vi "HFRR ADV v040 new software.vi"() -> ()   [LabVIEW 2025] (continued)
            n2157 = Bundle "Bundle"(w2313, w2312) -> (w2319:cluster{dbl[], dbl[]})  [unwired: 1 in]
            n2158 = Bundle "Bundle"(w2313, w2345) -> (w2456:cluster{dbl[], dbl[]})  [unwired: 1 in]
            n2159 = Bundle "Bundle"(w2313, w2341) -> (w2379:cluster{dbl[], dbl[]})  [unwired: 1 in]
            n2160 = Bundle "Bundle"(w2313, w2395) -> (w2403:cluster{dbl[], dbl[]})  [unwired: 1 in]
            n2161 = Bundle "Bundle"(w2313, w2397) -> (w2465:cluster{dbl[], dbl[]})  [unwired: 1 in]
            n2162 = Bundle "Bundle"(w2313, w2434) -> (w2447:cluster{dbl[], dbl[]})  [unwired: 1 in]
            n2163 = Bundle "Bundle"(w2343, w2339) -> (w2351:cluster{dbl[], dbl[]})  [unwired: 1 in]
            n2164 = Bundle "Bundle"(w2309, w2308) -> (w2317:cluster{dbl[], dbl[]})  [unwired: 1 in]
            n2165 = Bundle "Bundle"(w2309, w2343) -> (w2455:cluster{dbl[], dbl[]})  [unwired: 1 in]
            n2166 = Bundle "Bundle"(w2309, w2339) -> (w2377:cluster{dbl[], dbl[]})  [unwired: 1 in]
            n2167 = Bundle "Bundle"(w2309, w2393) -> (w2401:cluster{dbl[], dbl[]})  [unwired: 1 in]
            n2168 = Bundle "Bundle"(w2309, w2398) -> (w2463:cluster{dbl[], dbl[]})  [unwired: 1 in]
            n2169 = Bundle "Bundle"(w2309, w2416) -> (w2448:cluster{dbl[], dbl[]})  [unwired: 1 in]
            n2170 = call-poly <vilib>:"Mean.vi"("X"=w2396) -> ("mean"=→"CP1":dbl)  [unwired: 1 out]
            n2171 = call-poly <vilib>:"Mean.vi"("X"=w2337) -> ("mean"=→"КОФ2 3":dbl)  [unwired: 1 out]
            n2172 = call-poly <vilib>:"Mean.vi"("X"=w2395) -> ("mean"=→"CP2":dbl)  [unwired: 1 out]
            n2173 = call-poly <vilib>:"Mean.vi"("X"=w2397) -> ("mean"=→"КОФ2":dbl)  [unwired: 1 out]
            n2174 = call-poly <vilib>:"Mean.vi"("X"=w2335) -> ("mean"=→"КОФ2 5":dbl)  [unwired: 1 out]
            n2175 = call-poly <vilib>:"Mean.vi"("X"=w2393) -> ("mean"=→"CP4":dbl)  [unwired: 1 out]
            n2176 = call-poly <vilib>:"Mean.vi"("X"=w2398) -> ("mean"=→"КОФ4":dbl)  [unwired: 1 out]
            n2177 = Bundle "Bundle"(w2315, w2342) -> (w2306:cluster{dbl[], dbl[]})  [unwired: 1 in]
            n2178 = Bundle "Bundle"(w2315, w2396) -> (w2329:cluster{dbl[], dbl[]})  [unwired: 1 in]
            n2179 = Build Array "Build Array"(w2306, w2329) -> (w2332:cluster{dbl[], dbl[]}[])
            "XY Graph 17" <- w2332
            n2180 = Build Array "Build Array"(w2320, w2319, w2318, w2317) -> (→"Frequency ( Hz )":cluster{dbl[], dbl[]}[])
            n2181 = Build Array "Build Array"(w2348, w2349, w2350, w2351) -> (→"Air Temp ( °C ) vs Humidity ( % RH )":cluster{dbl[], dbl[]}[])
            n2182 = Build Array "Build Array"(w2333, w2456, w2454, w2455) -> (→"Air Temperature  ( °C )":cluster{dbl[], dbl[]}[])
            n2183 = Build Array "Build Array"(w2306, w2379, w2378, w2377) -> (→"Humidity ( %RH )":cluster{dbl[], dbl[]}[])
            n2184 = Build Array "Build Array"(w2334, w2465, w2464, w2463) -> (→"Coefficient Of Friction":cluster{dbl[], dbl[]}[])
            n2185 = Build Array "Build Array"(w2329, w2403, w2402, w2401) -> (→"Sample Temperature ( °C )":cluster{dbl[], dbl[]}[])
            n2186 = Build Array "Build Array"(w2307, w2447, w2449, w2448) -> (→"XY Graph 13":cluster{dbl[], dbl[]}[])
            n2187 = Bundle "Bundle"(w2315, w2338) -> (w2360:cluster{dbl[], dbl[]})  [unwired: 1 in]
            n2188 = Bundle "Bundle"(w2311, w2336) -> (w2358:cluster{dbl[], dbl[]})  [unwired: 1 in]
            n2189 = Bundle "Bundle"(w2313, w2337) -> (w2359:cluster{dbl[], dbl[]})  [unwired: 1 in]
            n2190 = Bundle "Bundle"(w2309, w2335) -> (w2357:cluster{dbl[], dbl[]})  [unwired: 1 in]
            n2191 = Build Array "Build Array"(w2360, w2359, w2358, w2357) -> (→"Stroke ( mm )":cluster{dbl[], dbl[]}[])
            n2192 = local write "XY Graph 16"(w2332) -> ()
          }
          frame #2 {
          }
          frame #3 {
            n2193 = local write "Numeric 8"(0 ("Numeric 8")) -> ()
            n2194 = local write "Numeric 11"(0 ("Numeric 11")) -> ()
            n2195 = local write "Numeric 12"(0 ("Numeric 12")) -> ()
            n2196 = local write "Numeric 13"(0 ("Numeric 13")) -> ()
            n2197 = property on="OPEN" class="Bool (strict)"("Visible"=TRUE) -> ()  [unwired: 2 in, 2 out]
            n2198 = local read "String Control 2"() -> (w2632:string)
            n2199 = local read "String Control 4"() -> (w2631:string)
            n2200 = local read "String Control 6"() -> (w2630:string)
            n2201 = local read "String Control 8"() -> (w2629:string)
            n2202 = Match Pattern(string=w2632, regular expression="Samples / cycle :- ") -> (after substring=w2646:string)  [unwired: 1 in, 3 out]
            n2203 = Match Pattern(string=w2632, regular expression="Frequency :- ") -> (after substring=w2665:string)  [unwired: 1 in, 3 out]
            n2204 = Match Pattern(string=w2631, regular expression="Samples / cycle :- ") -> (after substring=w2642:string)  [unwired: 1 in, 3 out]
            n2205 = Match Pattern(string=w2631, regular expression="Frequency :- ") -> (after substring=w2660:string)  [unwired: 1 in, 3 out]
            n2206 = Match Pattern(string=w2630, regular expression="Samples / cycle :- ") -> (after substring=w2638:string)  [unwired: 1 in, 3 out]
            n2207 = Match Pattern(string=w2630, regular expression="Frequency :- ") -> (after substring=w2655:string)  [unwired: 1 in, 3 out]
            n2208 = Match Pattern(string=w2629, regular expression="Samples / cycle :- ") -> (after substring=w2634:string)  [unwired: 1 in, 3 out]
            n2209 = Match Pattern(string=w2629, regular expression="Frequency :- ") -> (after substring=w2650:string)  [unwired: 1 in, 3 out]
            n2210 = String Subset(string=w2646, length (rest)=6 ("length (rest)")) -> (substring=w2648:string)  [unwired: 1 in]
            n2211 = String Subset(string=w2665, length (rest)=9 ("length (rest)")) -> (substring=w2667:string)  [unwired: 1 in]
            n2212 = String Subset(string=w2642, length (rest)=6 ("length (rest)")) -> (substring=w2644:string)  [unwired: 1 in]
            n2213 = String Subset(string=w2660, length (rest)=9 ("length (rest)")) -> (substring=w2662:string)  [unwired: 1 in]
            n2214 = String Subset(string=w2638, length (rest)=6 ("length (rest)")) -> (substring=w2640:string)  [unwired: 1 in]
            n2215 = String Subset(string=w2655, length (rest)=9 ("length (rest)")) -> (substring=w2657:string)  [unwired: 1 in]
            n2216 = String Subset(string=w2634, length (rest)=6 ("length (rest)")) -> (substring=w2636:string)  [unwired: 1 in]
            n2217 = String Subset(string=w2650, length (rest)=9 ("length (rest)")) -> (substring=w2652:string)  [unwired: 1 in]
            n2218 = Fract/Exp String To Number(string=w2648) -> (number=w2628:dbl)  [unwired: 3 in, 1 out]
            n2219 = Fract/Exp String To Number(string=w2667) -> (number=w2668:dbl)  [unwired: 3 in, 1 out]
            n2220 = Fract/Exp String To Number(string=w2644) -> (number=w2627:dbl)  [unwired: 3 in, 1 out]
            n2221 = Fract/Exp String To Number(string=w2662) -> (number=w2663:dbl)  [unwired: 3 in, 1 out]
            n2222 = Fract/Exp String To Number(string=w2640) -> (number=w2626:dbl)  [unwired: 3 in, 1 out]
            n2223 = Fract/Exp String To Number(string=w2657) -> (number=w2658:dbl)  [unwired: 3 in, 1 out]
            n2224 = Fract/Exp String To Number(string=w2636) -> (number=w2625:dbl)  [unwired: 3 in, 1 out]
            n2225 = Fract/Exp String To Number(string=w2652) -> (number=w2653:dbl)  [unwired: 3 in, 1 out]
            n2226 = local write "sample1"(w2628) -> ()
            n2227 = local write "freq1"(w2668) -> ()
            n2228 = local write "sample2"(w2627) -> ()
            n2229 = local write "freq2"(w2663) -> ()
            n2230 = local write "sample3"(w2626) -> ()
            n2231 = local write "freq3"(w2658) -> ()
            n2232 = local write "sample4"(w2625) -> ()
            n2233 = local write "freq 4"(w2653) -> ()
          }
        }
      }
    }
    n2234 = case shown="True" w2226 {
      selector: w2226 -> [_ w2245]
      frame False {
      }
      frame True {
        n2235 = Not(x=w2245) -> (.not. x?=w2241:bool)
        n2236 = local write "service 3"(w2241) -> ()
        n2237 = local write "OPEN 6"(w2241) -> ()
        n2238 = call <vilib>:"System Exec.vi"("wait until completion? (T)"=TRUE, "command line"="C:\\LAB-IQ\\Scar View.exe") -> ("error out"=→"error out 5":errorcluster)  [unwired: 6 in, 3 out]
      }
    }
    n2239 = case shown="\"Acquire\", Default" w2235 {
      frame "Acquire", Default {
        # "Elapsed time\ncof\nstroke\nAir temp\nTemp\nHumidity"
        n2240 = disable-structure shown="Disabled" {
          frame Disabled {
            n2241 = local read "Flag"() -> (w2944:dbl)
            n2242 = local read "RUN"() -> (w2941:bool)
            n2243 = Not(x=w2941) -> (.not. x?=w2940:bool)
            n2244 = Equal?(x=w2944, y=10.0) -> (x = y?=w2942:bool)
            n2245 = And(x=w2942, y=w2940) -> (x .and. y?=w2939:bool)
            n2246 = case shown="True" w2939 {
              frame False {
              }
              frame True {
                w2945 = FALSE ("Heater Button")
                n2247 = local write "Humidity"(w2945) -> ()
                n2248 = local write "Heater Button"(w2945) -> ()
              }
            }
          }
          frame Enabled {
          }
        }
        n2249 = disable-structure shown="Disabled" {
          frame Disabled {
            n2250 = case shown="True" {
              selector: _ -> [_ _]
              frame False {
              }
              frame True {
                w2994 = TRUE ("Heater")
                n2251 = local write "Humidity"(w2994) -> ()
                n2252 = local write "Heater Button"(w2994) -> ()
                n2253 = local read "TEST STANDARD"() -> (w2997:T3)
                n2254 = local read "TEST STANDARD"() -> (w2992:T3)
                n2255 = Equal?(x=w2997, y=enum16{"ASTM D6079", "ISO 12156", "Custom"}."ISO 12156" ("Test Standard")) -> (x = y?=w2995:bool)
                n2256 = Equal?(x=w2992, y=enum16{"ASTM D6079", "ISO 12156", "Custom"}."ASTM D6079" ("Test Standard")) -> (x = y?=w2991:bool)
                n2257 = case shown="True" w2995 {
                  frame False {
                  }
                  frame True {
                    n2258 = local write "airtempflg"(FALSE ("airtempflg")) -> ()
                    n2259 = local write item#-1(TRUE ("Heater")) -> ()
                  }
                }
                n2260 = case shown="True" w2991 {
                  frame False {
                  }
                  frame True {
                    n2261 = local write "airtempflg"(TRUE ("airtempflg")) -> ()
                    n2262 = local write item#-1(FALSE ("Heater")) -> ()
                  }
                }
              }
            }
          }
          frame Enabled {
          }
        }
        n2263 = stacked-sequence {
          frame #0 {
            n2264 = case shown="True" "RST FF" {
              frame False {
              }
              frame True {
                w3011 = 0.0 ("X Scale.Range:Maximum")
                n2265 = property on="Frictional Force ( N )" class="WFChart (strict)"("XScale.Maximum"=600.0 ("X Scale.Range:Maximum"), "XScale.Minimum"=w3011, "YScale.Maximum"=10.0 ("Y Scale.Range:Maximum"), "YScale.Minimum"=w3011) -> ()  [unwired: 2 in, 2 out]
              }
            }
          }
          frame #1 {
            n2266 = case shown="True" "RST TEMP" {
              frame False {
              }
              frame True {
                n2267 = property on="Temperature ( Deg C )" class="WFChart (strict)"("XScale.Minimum"=0.0 ("X Scale.Range:Minimum"), "XScale.Maximum"=600.0 ("X Scale.Range:Maximum"), "YScale.Minimum"=0.0 ("Y Scale.Range:Minimum"), "YScale.Maximum"=100.0 ("Y Scale.Range:Maximum")) -> ()  [unwired: 2 in, 2 out]
              }
            }
          }
          frame #2 {
            n2268 = case shown="True" "RSTCOF" {
              frame False {
              }
              frame True {
                n2269 = property on="Coefficient of Friction" class="WFChart (strict)"("XScale.Minimum"=0.0 ("X Scale.Range:Minimum"), "XScale.Maximum"=600.0 ("X Scale.Range:Maximum"), "YScale.Maximum"=1.0 ("X Scale.Range:Minimum"), "YScale.Minimum"=0.0 ("X Scale.Range:Minimum")) -> ()  [unwired: 2 in, 2 out]
              }
            }
          }
          frame #3 {
            n2270 = case shown="True" "RSTCOF 2" {
              frame False {
              }
              frame True {
                (unwired) 100.0 ("Y Scale.Range:Maximum")
                (unwired) 0.0 ("Y Scale.Range:Minimum")
                (unwired) 600.0 ("X Scale.Range:Maximum")
                (unwired) 0.0 ("X Scale.Range:Minimum")
              }
            }
          }
          frame #4 {
            n2271 = case shown="True" "RSTCOF 3" {
              frame False {
              }
              frame True {
                n2272 = property on="Electrical Contact Resistance ( % )" class="WFChart (strict)"("XScale.Minimum"=0.0 ("X Scale.Range:Minimum"), "XScale.Maximum"=600.0 ("X Scale.Range:Maximum"), "YScale.Minimum"=0.0 ("Y Scale.Range:Minimum"), "YScale.Maximum"=100.0 ("Y Scale.Range:Maximum")) -> ()  [unwired: 2 in, 2 out]
              }
            }
          }
        }
        n2273 = local read "RUN"() -> (w2934:bool)
        n2274 = case shown="False" w2934 {
          frame False {
          }
          frame True {
          }
        }
        n2275 = local read "RUN"() -> (w2938:bool)
        n2276 = case shown="False" w2938 {
          tunnel: [FALSE ("TEST RUNNING") TRUE ("TEST RUNNING")] -> w2937
          frame False {
            w3030 = 0.0 ("Flag")
            n2277 = local write "Elapsed time"(0.0 ("elapsedtime")) -> ()
            n2278 = local write "Time Remaining"(w3030) -> ()
            n2279 = local write "Flag"(w3030) -> ()
            n2280 = local write "Remaining Time"(w3030) -> ()
          }
          frame True {
            n2281 = local write "Flag"(10.0 ("Flag")) -> ()
          }
        }
        n2282 = local read "AIR TEMP"() -> (w2932:dbl)
        n2283 = Greater Or Equal?(x=w2932, y=15.0) -> (x >= y?=w2933:bool)
        "powstat" <- w2933
        n2284 = case shown="True" "Save & Continue" {
          frame False {
          }
          frame True {
            n2285 = local read "USER ID"() -> (w3339:string)
            n2286 = local read "FILE"() -> (w3347:string)
            n2287 = String Length(string=w3347) -> (length=w3345:i32)
            n2288 = String Length(string=w3339) -> (length=w3342:i32)
            n2289 = Greater?(x=w3345, y=0) -> (0:w3344:bool)
            n2290 = Greater?(x=w3342, y=0) -> (0:w3341:bool)
            n2291 = And(x=w3344, y=w3341) -> (x .and. y?=w3340:bool)
            n2292 = case shown="True" w3340 {
              frame False {
                n2293 = stacked-sequence {
                  frame #0 {
                    n2294 = One Button Dialog(message="Please Enter a File Name and Operator ID to save data !", button name ("OK")="Ok") -> ()  [unwired: 1 out]
                  }
                  frame #1 {
                    n2295 = local write "Save & Continue"(FALSE ("OK Button")) -> ()
                  }
                }
                n2296 = local write "Save & Continue"(FALSE ("OK Button")) -> ()
              }
              frame True {
                n2297 = stacked-sequence {
                  frame #0 {
                    n2298 = local read "FILE"() -> (w3353:string)
                    n2299 = call "file check.vi"("file name in"=w3353) -> ("file name out"=w3352:string)  [unwired: 9 in, 1 out]
                    n2300 = call <vilib>:"Application Directory.vi"() -> ("Application Directory"=w3363:path)
                    n2301 = Build Path(base path=w3363, name or relative path="data") -> (appended path=w3362:path)
                    n2302 = call <vilib>:"Trim Whitespace.vi"("string"=w3352) -> ("trimmed string"=w3360:string)  [unwired: 1 in]
                    n2303 = call <vilib>:"Trim Whitespace.vi"("string"=w3352) -> ("trimmed string"=w3361:string)  [unwired: 1 in]
                    n2304 = List Folder(path=w3362) -> (folder names=w3358:string[])  [unwired: 3 in, 3 out]
                    n2305 = Match Pattern(string=w3360, regular expression="_(") -> (before substring=w3357:string)  [unwired: 1 in, 3 out]
                    n2306 = for {
                      tunnel: w3358 -> [w3372] mode=indexing
                      tunnel: w3357 -> [w3370]
                      shift-right: [w3368] -> w3355
                      shift-left: bool[] [] -> [w3369]
                      n2307 = Match Pattern(string=w3372, regular expression="_(") -> (before substring=w3371:string)  [unwired: 1 in, 3 out]
                      n2308 = Equal?(x=w3371, y=w3370) -> (x = y?=w3367:bool)
                      n2309 = case shown="True" w3367 {
                        tunnel: w3367 -> [_ w3375]
                        tunnel: w3369 -> [w3374 w3377]
                        tunnel: [w3374 w3376] -> w3368
                        frame False {
                        }
                        frame True {
                          n2310 = Insert Into Array(array=w3377, new element=w3375) -> (w3376:bool[])  [unwired: 1 in]
                        }
                      }
                    }
                    n2311 = Equal?(x=w3358, y=w3357) -> (x = y?=w3366:bool[])
                    n2312 = Or Array Elements(Boolean array=w3366) -> (logical OR=w3365:bool)
                    n2313 = Array Size(array=w3355) -> (size(s)=w3354:i32)
                    n2314 = case shown="True" w3365 {
                      tunnel: w3361 -> [_ w3385]
                      tunnel: w3354 -> [_ w3378]
                      frame False {
                      }
                      frame True {
                        n2315 = Number To Decimal String(number=w3378) -> (decimal integer string=w3381:string)  [unwired: 1 in]
                        n2316 = Search/Split String(string=w3385, search string/char (-)="_(" ("regular expression")) -> (substring before match=w3383:string)  [unwired: 1 in, 2 out]
                        n2317 = Concatenate Strings(w3383, "_(" ("regular expression"), w3381, ")" ("regular expression")) -> (w3379:string)
                        n2318 = local write "FILE"(w3379) -> ()
                      }
                    }
                  }
                  frame #1 {
                    w3388 = 0.0
                    w3401 = cluster{"y":dbl, dbl, "y":dbl}[] [] ("History Data")
                    w3402 = FALSE ("Heater Button")
                    (unwired) ")!" ("string")
                    (unwired) ")" ("string")
                    w3400 = dbl[] [] ("History Data")
                    w3406 = "\r"
                    # "C:\\WinDucom\\Data\\"
                    # "C:\\LAB-IQ-NXT\\data"
                    n2319 = local write "Humidity ( %RH )"(w3388) -> ()
                    n2320 = local write "Frequency ( Hz )"(w3388) -> ()
                    n2321 = local write "Stroke 3"(w3388) -> ()
                    n2322 = local write "speedop"(0.0 ("PIDclk 2")) -> ()
                    n2323 = local write "Set Temp 2"(65.0 ("Set Temp 2")) -> ()
                    n2324 = local write "AIR TEMP"(w3388) -> ()
                    n2325 = local write "clk"(0.0 ("clk")) -> ()
                    n2326 = local write "Stroke 4"(w3388) -> ()
                    n2327 = local write "COF 2"(w3388) -> ()
                    n2328 = local write "TEMP"(w3388) -> ()
                    n2329 = local write "ecr 3"(w3388) -> ()
                    n2330 = local write "FF 3"(w3388) -> ()
                    n2331 = local write "FF 2"(w3388) -> ()
                    n2332 = property on="Humidity ( %RH ) 2" class="WFChart (strict)"("History Data"=w3400) -> ()  [unwired: 2 in, 2 out]
                    n2333 = property on="Coefficient of Friction" class="WFChart (strict)"("History Data"=w3400) -> ()  [unwired: 2 in, 2 out]
                    n2334 = property on="Coefficient of Friction" class="WFChart (strict)"("History Data"=w3400) -> ()  [unwired: 2 in, 2 out]
                    n2335 = property on="Frictional Force ( N )" class="WFChart (strict)"("History Data"=w3400) -> ()  [unwired: 2 in, 2 out]
                    n2336 = property on="Electrical Contact Resistance ( % )" class="WFChart (strict)"("History Data"=w3400) -> ()  [unwired: 2 in, 2 out]
                    n2337 = property on="Electrical Contact Resistance ( % )" class="WFChart (strict)"("History Data"=w3400) -> ()  [unwired: 2 in, 2 out]
                    n2338 = property on="Temperature ( Deg C )" class="WFChart (strict)"("History Data"=w3400) -> ()  [unwired: 2 in, 2 out]
                    n2339 = property on="Frictional Force ( N )" class="WFChart (strict)"("History Data"=w3400) -> ()  [unwired: 2 in, 2 out]
                    n2340 = property on="Coefficient of Friction" class="WFChart (strict)"("History Data"=w3400) -> ()  [unwired: 2 in, 2 out]
                    n2341 = property on="Frictional Force ( N )" class="WFChart (strict)"("History Data"=w3400) -> ()  [unwired: 2 in, 2 out]
                    n2342 = property on="Electrical Contact Resistance ( % )" class="WFChart (strict)"("History Data"=w3400) -> ()  [unwired: 2 in, 2 out]
                    n2343 = property on="Temperature ( Deg C )" class="WFChart (strict)"("History Data"=w3400) -> ()  [unwired: 2 in, 2 out]
                    n2344 = property on="Stroke ( mm )" class="WFChart (strict)"("History Data"=w3401) -> ()  [unwired: 2 in, 2 out]
                    n2345 = property on="Stroke ( mm )" class="WFChart (strict)"("History Data"=w3401) -> ()  [unwired: 2 in, 2 out]
                    n2346 = local write "Humidity"(w3402) -> ()
                    n2347 = local write "Heater Button"(w3402) -> ()
                    n2348 = local read "FILE"() -> (w3396:string)
                    n2349 = disable-structure shown="Enabled" {
                      disable-tunnel: [w3440 _] -> w3387
                      frame Enabled {
                        n2350 = local read "NORMAL LOAD"() -> (w3440:dbl)
                      }
                      frame Disabled {
                      }
                    }
                    n2351 = call "file check.vi"("file name in"=w3396) -> ("error out"=w3399:errorcluster, "file name out"=w3393:string)  [unwired: 9 in]
                    n2352 = call "FILE PATH CREATION.vi"("error in"=w3399, "FILE NAME :"=w3393) -> ("FILE OUT"=w3392:path)  [unwired: 8 in, 1 out]
                    n2353 = Concatenate Strings(w3393, ".dgf" ("Substring")) -> (w3398:string)
                    n2354 = Concatenate Strings(w3393, ".duf" ("Substring")) -> (w3394:string)
                    n2355 = Multiply(x=w3387, y=1.0) -> (x*y=w3419:dbl)
                    n2356 = Build Path(base path=w3392, name or relative path=w3398) -> (appended path=w3391:path)
                    n2357 = Build Path(base path=w3392, name or relative path=w3394) -> (appended path=w3390:path)
                    n2358 = Number To Fractional String(number=w3419, width (-)=i16 5, precision (6)=i16 2) -> (F-format string=w3427:string)  [unwired: 1 in]
                    n2359 = local read "tested by"() -> (w3386:string)
                    n2360 = local read "Fuel Discription :"() -> (w3415:string)
                    n2361 = local read "Batch Ref Num :"() -> (w3404:string)
                    n2362 = Get Date/Time String(date format (0)=enum16{"short", "long", "abbreviated"}."short") -> (date string=w3438:string, time string=w3435:string)  [unwired: 2 in]
                    n2363 = local read "Remarks :"() -> (w3414:string)
                    n2364 = Concatenate Strings("Load :- " ("Substring"), w3427, " grams ," ("Substring")) -> (w3426:string)
                    n2365 = local read "String 41"() -> (w3407:string)
                    n2366 = Concatenate Strings(w3415) -> (w3416:string)
                    n2367 = Concatenate Strings(w3404) -> (w3403:string)
                    n2368 = Concatenate Strings(w3386) -> (w3410:string)
                    n2369 = Concatenate Strings("(" ("Substring"), w3438, ")" ("Substring"), w3435) -> (w3409:string)
                    "concatenated string" <- w3409
                    n2370 = Concatenate Strings(w3414, "," ("string")) -> (w3413:string)
                    n2371 = Concatenate Strings("  TIME;      COF;       STROKE;     AIR TEMP;  TEMP;  HUMIDITY;  ECR; PID-OUT; FREQUENCY" ("Substring"), "\r") -> (w3422:string)
                    n2372 = Concatenate Strings(w3407, w3406, "Fuel Discription :-" ("Substring"), w3416, w3406, w3426, w3406, "Batch Ref Num :-" ("Substring"), w3403, w3406, " Remarks :- " ("Substring"), w3413, w3406, " Date :- " ("Substring"), w3409, w3406, "Tested By :-" ("Substring"), w3410) -> (w3420:string)
                    "REMARKS" <- w3420
                    n2373 = call <vilib>:"Write Characters To File.vi"("append to file? (new file:F)"=FALSE, "character string"=w3422, "file path (dialog if empty)"=w3391) -> ()  [unwired: 2 in, 1 out]
                    n2374 = call <vilib>:"Write Characters To File.vi"("append to file? (new file:F)"=FALSE, "character string"=w3420, "file path (dialog if empty)"=w3390) -> ()  [unwired: 2 in, 1 out]
                  }
                  frame #2 {
                    n2375 = local write "Cycles elapsed"(0 ("Cycles elapsed")) -> ()
                    n2376 = local write "cyclecount"(0 ("cyclecount")) -> ()
                    n2377 = local write "Save & Continue"(FALSE ("OK")) -> ()
                    n2378 = local write "autostrtflg"(TRUE ("autostrtflg")) -> ()
                    n2379 = local write "Save"(FALSE ("Save")) -> ()
                    n2380 = Get Date/Time In Seconds() -> (seconds since 1Jan1904=w3445:timestamp)
                    n2381 = To Double Precision Float(number=w3445) -> (double precision float=w3444:dbl)
                    n2382 = local write "acq timer"(w3444) -> ()
                    n2383 = One Button Dialog(message="Please ensure sample is mounted properly and machine is ready in all aspects for testing !", button name ("OK")="Ok") -> ()  [unwired: 1 out]
                  }
                  frame #3 {
                    n2384 = stacked-sequence {
                      frame #0 {
                        n2385 = local write "Main Dashboard Buttons"(T1."Dashboard" ("Main Dashboard Buttons")) -> ()
                        n2386 = local write "Main Tab"(T2."Acquire" ("Main Tab")) -> ()
                      }
                      frame #1 {
                        n2387 = local write "EVENT LOG"("" ("EVENT LOG")) -> ()
                      }
                      frame #2 {
                        n2388 = Wait (ms)(milliseconds to wait=u32 50) -> ()  [unwired: 1 out]
                      }
                      frame #3 {
                        n2389 = disable-structure shown="Disabled" {
                          frame Disabled {
                            n2390 = local read "EVENT LOG"() -> (w3457:string)
                            n2391 = call "Event Log.vi"("Content"="Test Details", "EVENT LOG"=w3457) -> ("EVENT LOG"=w3456:string)  [unwired: 8 in, 1 out]
                            n2392 = local write "EVENT LOG"(w3456) -> ()
                          }
                          frame Enabled {
                          }
                        }
                      }
                      frame #4 {
                        n2393 = Wait (ms)(milliseconds to wait=u32 50) -> ()  [unwired: 1 out]
                      }
                      frame #5 {
                        n2394 = local read "FILE"() -> (w3459:string)
                        n2395 = Concatenate Strings("File Name :" ("Content"), w3459) -> (w3460:string)
                        n2396 = local read "EVENT LOG"() -> (w3463:string)
                        n2397 = call "Event Log.vi"("Content"=w3460, "EVENT LOG"=w3463) -> ("EVENT LOG"=w3462:string)  [unwired: 8 in, 1 out]
                        n2398 = local write "EVENT LOG"(w3462) -> ()
                      }
                      frame #6 {
                        n2399 = Wait (ms)(milliseconds to wait=u32 50) -> ()  [unwired: 1 out]
                      }
                      frame #7 {
                        n2400 = local read "Batch Ref Num :"() -> (w3465:string)
                        n2401 = Concatenate Strings("Batch Ref No :" ("Content"), w3465) -> (w3466:string)
                        n2402 = local read "EVENT LOG"() -> (w3469:string)
                        n2403 = call "Event Log.vi"("Content"=w3466, "EVENT LOG"=w3469) -> ("EVENT LOG"=w3468:string)  [unwired: 8 in, 1 out]
                        n2404 = local write "EVENT LOG"(w3468) -> ()
                      }
                      frame #8 {
                        n2405 = Wait (ms)(milliseconds to wait=u32 50) -> ()  [unwired: 1 out]
                      }
                      frame #9 {
                        n2406 = local read "tested by"() -> (w3471:string)
                        n2407 = Concatenate Strings("Tested By :" ("Content"), w3471) -> (w3472:string)
                        n2408 = local read "EVENT LOG"() -> (w3475:string)
                        n2409 = call "Event Log.vi"("Content"=w3472, "EVENT LOG"=w3475) -> ("EVENT LOG"=w3474:string)  [unwired: 8 in, 1 out]
                        n2410 = local write "EVENT LOG"(w3474) -> ()
                      }
                      frame #10 {
                        n2411 = Wait (ms)(milliseconds to wait=u32 50) -> ()  [unwired: 1 out]
                      }
                      frame #11 {
                        n2412 = local read "TEST STANDARD"() -> (w3478:T3)
                        n2413 = case shown="\"ASTM D6079\", Default" w3478 {
                          tunnel: ["ASTM D6079" "ISO 12156" "CEC F-096-A-06" "Custom"] -> w3477
                          frame "ASTM D6079", Default {
                          }
                          frame "ISO 12156" {
                          }
                          frame "CEC F-096-A-06" {
                          }
                          frame "Custom" {
                          }
                        }
                        n2414 = Concatenate Strings("Test Standard :" ("Content"), w3477) -> (w3479:string)
                        n2415 = local read "EVENT LOG"() -> (w3482:string)
                        n2416 = call "Event Log.vi"("Content"=w3479, "EVENT LOG"=w3482) -> ("EVENT LOG"=w3481:string)  [unwired: 8 in, 1 out]
                        n2417 = local write "EVENT LOG"(w3481) -> ()
                      }
                      frame #12 {
                        n2418 = Wait (ms)(milliseconds to wait=u32 50) -> ()  [unwired: 1 out]
                      }
                      frame #13 {
                        n2419 = local read "Fuel Discription :"() -> (w3488:string)
                        n2420 = Concatenate Strings("Fuel Description :" ("Content"), w3488) -> (w3489:string)
                        n2421 = local read "EVENT LOG"() -> (w3492:string)
                        n2422 = call "Event Log.vi"("Content"=w3489, "EVENT LOG"=w3492) -> ("EVENT LOG"=w3491:string)  [unwired: 8 in, 1 out]
                        n2423 = local write "EVENT LOG"(w3491) -> ()
                      }
                      frame #14 {
                        n2424 = Wait (ms)(milliseconds to wait=u32 50) -> ()  [unwired: 1 out]
                      }
                      frame #15 {
                        n2425 = local read "Remarks :"() -> (w3494:string)
                        n2426 = Concatenate Strings("Remarks :" ("Content"), w3494) -> (w3495:string)
                        n2427 = local read "EVENT LOG"() -> (w3498:string)
                        n2428 = call "Event Log.vi"("Content"=w3495, "EVENT LOG"=w3498) -> ("EVENT LOG"=w3497:string)  [unwired: 8 in, 1 out]
                        n2429 = local write "EVENT LOG"(w3497) -> ()
                      }
                      frame #16 {
                        n2430 = Wait (ms)(milliseconds to wait=u32 50) -> ()  [unwired: 1 out]
                      }
                      frame #17 {
                        n2431 = local read "USER ID"() -> (w3500:string)
                        n2432 = Concatenate Strings("Operator ID :" ("Content"), w3500) -> (w3502:string)
                        n2433 = local read "EVENT LOG"() -> (w3504:string)
                        n2434 = call "Event Log.vi"("Content"=w3502, "EVENT LOG"=w3504) -> ("EVENT LOG"=w3503:string)  [unwired: 8 in, 1 out]
                        n2435 = local write "EVENT LOG"(w3503) -> ()
                      }
                      frame #18 {
                        n2436 = Wait (ms)(milliseconds to wait=u32 50) -> ()  [unwired: 1 out]
                      }
                      frame #19 {
                        n2437 = disable-structure shown="Disabled" {
                          frame Disabled {
                            n2438 = local read "EVENT LOG"() -> (w3508:string)
                            n2439 = call "Event Log.vi"("Content"="Test Parameter", "EVENT LOG"=w3508) -> ("EVENT LOG"=w3507:string)  [unwired: 8 in, 1 out]
                            n2440 = local write "EVENT LOG"(w3507) -> ()
                          }
                          frame Enabled {
                          }
                        }
                      }
                      frame #20 {
                        n2441 = Wait (ms)(milliseconds to wait=u32 50) -> ()  [unwired: 1 out]
                      }
                      frame #21 {
                        n2442 = local read "Set Hz"() -> (w3512:dbl)
                        n2443 = Number To Fractional String(number=w3512, precision (6)=i16 2) -> (F-format string=w3511:string)  [unwired: 2 in]
                        n2444 = Concatenate Strings("Set Frequency [Hz] :" ("Content"), w3511) -> (w3514:string)
                        n2445 = local read "EVENT LOG"() -> (w3516:string)
                        n2446 = call "Event Log.vi"("Content"=w3514, "EVENT LOG"=w3516) -> ("EVENT LOG"=w3515:string)  [unwired: 8 in, 1 out]
                        n2447 = local write "EVENT LOG"(w3515) -> ()
                      }
                      frame #22 {
                        n2448 = Wait (ms)(milliseconds to wait=u32 50) -> ()  [unwired: 1 out]
                      }
                      frame #23 {
                        n2449 = local read "NORMAL LOAD"() -> (w3519:dbl)
                        n2450 = Number To Fractional String(number=w3519, precision (6)=i16 2) -> (F-format string=w3520:string)  [unwired: 2 in]
                        n2451 = Concatenate Strings("Applied Load [grams] :" ("Content"), w3520) -> (w3522:string)
                        n2452 = local read "EVENT LOG"() -> (w3524:string)
                        n2453 = call "Event Log.vi"("Content"=w3522, "EVENT LOG"=w3524) -> ("EVENT LOG"=w3523:string)  [unwired: 8 in, 1 out]
                        n2454 = local write "EVENT LOG"(w3523) -> ()
                      }
                      frame #24 {
                        n2455 = Wait (ms)(milliseconds to wait=u32 50) -> ()  [unwired: 1 out]
                      }
                      frame #25 {
                        n2456 = local read "Set Strk"() -> (w3527:dbl)
                        n2457 = Number To Fractional String(number=w3527, precision (6)=i16 2) -> (F-format string=w3528:string)  [unwired: 2 in]
                        n2458 = Concatenate Strings("Set Stroke [mm] :" ("Content"), w3528) -> (w3530:string)
                        n2459 = local read "EVENT LOG"() -> (w3532:string)
                        n2460 = call "Event Log.vi"("Content"=w3530, "EVENT LOG"=w3532) -> ("EVENT LOG"=w3531:string)  [unwired: 8 in, 1 out]
                        n2461 = local write "EVENT LOG"(w3531) -> ()
                      }
                      frame #26 {
                        n2462 = Wait (ms)(milliseconds to wait=u32 50) -> ()  [unwired: 1 out]
                      }
                      frame #27 {
                        n2463 = local read "Set Temp"() -> (w3535:dbl)
                        n2464 = Number To Fractional String(number=w3535, precision (6)=i16 2) -> (F-format string=w3536:string)  [unwired: 2 in]
                        n2465 = Concatenate Strings("Set Temperature [deg C] :" ("Content"), w3536) -> (w3538:string)
                        n2466 = local read "EVENT LOG"() -> (w3540:string)
                        n2467 = call "Event Log.vi"("Content"=w3538, "EVENT LOG"=w3540) -> ("EVENT LOG"=w3539:string)  [unwired: 8 in, 1 out]
                        n2468 = local write "EVENT LOG"(w3539) -> ()
                      }
                      frame #28 {
                        n2469 = Wait (ms)(milliseconds to wait=u32 50) -> ()  [unwired: 1 out]
                      }
                      frame #29 {
                        n2470 = local read "Set Rh"() -> (w3543:dbl)
                        n2471 = Number To Fractional String(number=w3543, precision (6)=i16 2) -> (F-format string=w3544:string)  [unwired: 2 in]
                        n2472 = Concatenate Strings("Set Humidity [%RH] :" ("Content"), w3544) -> (w3546:string)
                        n2473 = local read "EVENT LOG"() -> (w3548:string)
                        n2474 = call "Event Log.vi"("Content"=w3546, "EVENT LOG"=w3548) -> ("EVENT LOG"=w3547:string)  [unwired: 8 in, 1 out]
                        n2475 = local write "EVENT LOG"(w3547) -> ()
                      }
                      frame #30 {
                        n2476 = Wait (ms)(milliseconds to wait=u32 50) -> ()  [unwired: 1 out]
                      }
                      frame #31 {
                        n2477 = local read "test time"() -> (w3551:dbl)
                        n2478 = Number To Fractional String(number=w3551, precision (6)=i16 1) -> (F-format string=w3552:string)  [unwired: 2 in]
                        n2479 = Concatenate Strings("Test Duration [mins] :" ("Content"), w3552) -> (w3554:string)
                        n2480 = local read "EVENT LOG"() -> (w3556:string)
                        n2481 = call "Event Log.vi"("Content"=w3554, "EVENT LOG"=w3556) -> ("EVENT LOG"=w3555:string)  [unwired: 8 in, 1 out]
                        n2482 = local write "EVENT LOG"(w3555) -> ()
                      }
                      frame #32 {
                        w3557 = dbl[] [] ("History Data")
                        w3558 = cluster{"y":dbl, dbl, "y":dbl}[] [] ("History Data")
                        w3559 = FALSE ("Visible")
                        n2483 = property on="Stroke ( mm )" class="WFChart (strict)"("History Data"=w3558) -> ()  [unwired: 2 in, 2 out]
                        n2484 = property on="Humidity ( %RH ) 2" class="WFChart (strict)"("History Data"=w3557) -> ()  [unwired: 2 in, 2 out]
                        n2485 = property on="Temperature ( Deg C )" class="WFChart (strict)"("History Data"=w3557) -> ()  [unwired: 2 in, 2 out]
                        n2486 = property on="Electrical Contact Resistance ( % )" class="WFChart (strict)"("History Data"=w3557) -> ()  [unwired: 2 in, 2 out]
                        n2487 = property on="Coefficient of Friction" class="WFChart (strict)"("History Data"=w3557) -> ()  [unwired: 2 in, 2 out]
                        n2488 = property on="Frictional Force ( N )" class="WFChart (strict)"("History Data"=w3557) -> ()  [unwired: 2 in, 2 out]
                        n2489 = property on="Coefficient of Friction" class="WFChart (strict)"("History Data"=w3557) -> ()  [unwired: 2 in, 2 out]
                        n2490 = property on="Frictional Force ( N )" class="WFChart (strict)"("History Data"=w3557) -> ()  [unwired: 2 in, 2 out]
                        n2491 = property on="Electrical Contact Resistance ( % )" class="WFChart (strict)"("History Data"=w3557) -> ()  [unwired: 2 in, 2 out]
                        n2492 = property on="Stroke ( mm )" class="WFChart (strict)"("History Data"=w3558) -> ()  [unwired: 2 in, 2 out]
                        n2493 = property on="Temperature ( Deg C )" class="WFChart (strict)"("History Data"=w3557) -> ()  [unwired: 2 in, 2 out]
                        n2494 = property on="Service Password Log" class="Str"("Visible"=w3559) -> ()  [unwired: 2 in, 2 out]
                        n2495 = property on="Password 3" class="Clust (strict)"("Visible"=w3559) -> ()  [unwired: 2 in, 2 out]
                      }
                    }
                    "TEST FILE NAM,E SAVED" <- TRUE ("TEST FILE NAM,E SAVED")
                  }
                }
              }
            }
          }
        }
        n2496 = local write "Test \nStatus"(w2937) -> ()
        n2497 = local write "Save"(w2937) -> ()
        n2498 = local read "Main Tab"() -> (w2931:T2)
        n2499 = case shown="True" w2934 {
          frame False {
            n2500 = local read "Rt 3"() -> (w3002:bool)
            n2501 = case shown="True" w3002 {
              frame False {
              }
              frame True {
                n2502 = local write "Rt 3"(FALSE ("Rt 3")) -> ()
              }
            }
            "Rt" <- TRUE ("Rt")
            "Rt 2" <- FALSE ("Rt")
          }
          frame True {
            n2503 = local read "Rt"() -> (w3008:bool)
            n2504 = local write "Rt 2"(TRUE ("Rt 2")) -> ()
            n2505 = case shown="True" w3008 {
              frame False {
              }
              frame True {
                n2506 = local write "Rt"(FALSE ("Rt")) -> ()
              }
            }
            "Rt 3" <- TRUE ("Rt 3")
          }
        }
        n2507 = case shown="\"Acquire\"" w2931 {
          tunnel: w2933 -> [_ w3037]
          frame Default {
            w3036 = 0.0 ("output")
            n2508 = local write "PID-out"(w3036) -> ()
            n2509 = local write "Frequency ( Hz )"(w3036) -> ()
            n2510 = local write "STROKE Initialize"(TRUE ("STROKE Initialize")) -> ()
          }
          frame "Acquire" {
            n2511 = stacked-sequence {
              frame #0 {
                n2512 = local read "Auto Start Test"() -> (w3039:bool)
                n2513 = case shown="True" w3039 {
                  tunnel: "RUN" -> [w3060 w3063]
                  tunnel: [w3060 w3062] -> w3040
                  frame False {
                  }
                  frame True {
                    n2514 = local read "Auto Start Temp"() -> (w3061:bool)
                    n2515 = Or(x=w3063, y=w3061) -> (x .or. y?=w3062:bool)
                  }
                }
                n2516 = local read "clk"() -> (w3059:dbl)
                n2517 = local read "Save"() -> (w3055:bool)
                n2518 = Equal?(x=w3059, y=0.0) -> (x = y?=w3056:bool)
                n2519 = And(x=w3056, y=w3055) -> (x .and. y?=w3057:bool)
                n2520 = Not(x="Engage") -> (.not. x?=w3046:bool)
                n2521 = case shown="False" w3040 {
                  tunnel: [0.0 w3086] -> w3042
                  frame False {
                    (unwired) TRUE ("Visible")
                    n2522 = local read "Auto Start Test"() -> (w3067:bool)
                    n2523 = local write "Start Time"(TRUE ("Start Time")) -> ()
                    n2524 = property on="Stroke 2" class="DigNum (strict)"("Visible"=FALSE) -> ()  [unwired: 2 in, 2 out]
                    n2525 = case shown="False" w3067 {
                      frame False {
                        n2526 = property on="Heater Button" class="Bool (strict)"("DisabledEnum"=T19."Enabled" ("Disabled")) -> ()  [unwired: 2 in, 2 out]
                        n2527 = property on="Humidity" class="Bool (strict)"("DisabledEnum"=T19."Enabled" ("Disabled")) -> ()  [unwired: 2 in, 2 out]
                      }
                      frame True {
                      }
                    }
                    n2528 = case shown="False" "TestCompFlg" {
                      frame False {
                        n2529 = local read "StartFlg"() -> (w3075:bool)
                        n2530 = case shown="True" w3075 {
                          frame False {
                          }
                          frame True {
                            n2531 = stacked-sequence {
                              frame #0 {
                                n2532 = local read "EVENT LOG"() -> (w3079:string)
                                n2533 = call "Event Log.vi"("Content"="Test was interrupted", "EVENT LOG"=w3079) -> ("EVENT LOG"=w3080:string)  [unwired: 8 in, 1 out]
                                n2534 = local write "EVENT LOG"(w3080) -> ()
                                n2535 = property on="RUN" class="Bool (strict)"("Visible"=TRUE) -> ()  [unwired: 2 in, 2 out]
                                n2536 = property on="Auto Start Test" class="Bool (strict)"("Visible"=TRUE) -> ()  [unwired: 2 in, 2 out]
                              }
                              frame #1 {
                                w3082 = FALSE ("StartFlg")
                                n2537 = property on="Heater Button" class="Bool (strict)"("Val(Sgnl)"=FALSE ("Value (Signaling)")) -> ()  [unwired: 2 in, 2 out]
                                n2538 = local write "Heater Button"(w3082) -> ()
                                n2539 = local write "StartFlg"(w3082) -> ()
                                n2540 = local write "Humidity"(w3082) -> ()
                              }
                              frame #2 {
                                n2541 = local write "Due Write"("VC;0" ("Command")) -> ()
                              }
                              frame #3 {
                                n2542 = Wait (ms)(milliseconds to wait=u32 1500) -> ()  [unwired: 1 out]
                              }
                              frame #4 {
                                n2543 = local write "Due Write"("HE;0" ("Command")) -> ()
                              }
                            }
                          }
                        }
                      }
                      frame True {
                      }
                    }
                    n2544 = local write "String 14"("Test will autostart once parameters reach the set value." ("String 14")) -> ()
                  }
                  frame True {
                    (unwired) FALSE ("Visible")
                    n2545 = property on="Stroke 2" class="DigNum (strict)"("Visible"=TRUE) -> ()  [unwired: 2 in, 2 out]
                    n2546 = property on="STOP 2" class="Bool (strict)"("Disabled"=u8 2) -> ()  [unwired: 2 in, 2 out]
                    n2547 = local write "String 14"(" Running....." ("String 14")) -> ()
                    n2548 = property on="Heater Button" class="Bool (strict)"("DisabledEnum"=T19."Disabled and Grayed Out" ("Disabled")) -> ()  [unwired: 2 in, 2 out]
                    n2549 = property on="Humidity" class="Bool (strict)"("DisabledEnum"=T19."Disabled and Grayed Out" ("Disabled")) -> ()  [unwired: 2 in, 2 out]
                    n2550 = case shown="True" "Start Time" {
                      selector: "Start Time" -> [_ w3105]
                      frame False {
                      }
                      frame True {
                        n2551 = Not(x=w3105) -> (.not. x?=w3104:bool)
                        n2552 = local write "Start Time"(w3104) -> ()
                        n2553 = local read "EVENT LOG"() -> (w3106:string)
                        n2554 = call "Event Log.vi"("Content"="Test in progress", "EVENT LOG"=w3106) -> ("EVENT LOG"=w3108:string)  [unwired: 8 in, 1 out]
                        n2555 = local write "EVENT LOG"(w3108) -> ()
                      }
                    }
                    n2556 = disable-structure shown="Enabled" {
                      disable-tunnel: [w3097 w3103] -> w3086
                      frame Disabled {
                        n2557 = local read "Set Hz"() -> (w3100:dbl)
                        n2558 = call <vilib>:"Uniform White Noise Waveform.vi"() -> ("signal out"=w3099:waveform(dbl))  [unwired: 10 in, 1 out]
                        n2559 = Random Number (0-1)() -> (number: 0 to 1=w3096:dbl)
                        n2560 = Add(x=w3100, y=w3099) -> (x+y=w3098:waveform(dbl))
                        n2561 = Multiply(x=ext 0.01 ("y"), y=w3096) -> (x*y=w3094:ext)
                        n2562 = Multiply(x=w3098, y=w3094) -> (x*y=w3097:waveform(ext))
                      }
                      frame Enabled {
                        n2563 = call-poly <vilib>:"Random Number (Range).vi"("lower bound (0)"=49.89, "upper bound (100)"=50.8) -> ("number"=w3103:dbl)  [unwired: 9 in]
                      }
                    }
                    "StartFlg" <- TRUE ("StartFlg")
                  }
                }
                n2564 = case shown="True" w3057 {
                  frame False {
                  }
                  frame True {
                    n2565 = local write "clk"(10.0 ("clk")) -> ()
                    n2566 = Get Date/Time In Seconds() -> (seconds since 1Jan1904=w3111:timestamp)
                    n2567 = To Double Precision Float(number=w3111) -> (double precision float=w3109:dbl)
                    n2568 = local write "acq timer"(w3109) -> ()
                    n2569 = local write "act save time"(w3109) -> ()
                  }
                }
                n2570 = call "Elapsed Time"("Time Target (s)"="Countdown", "Reset"=w3046) -> ("Elapsed Time (s)"=w3051:dbl, "Time has Elapsed"=w3049:bool)  [unwired: 10 in, 6 out]
                "Countdown 2" <- w3051
                n2571 = Subtract(x=w3051, y=2.0) -> (x-y=w3054:dbl)
                n2572 = Less?(x=w3054, y="Countdown") -> (x < y?=w3052:bool)
                n2573 = And(x=w3052, y=w3049) -> (x .and. y?=w3048:bool)
                n2574 = case shown="True" w3048 {
                  frame False {
                  }
                  frame True {
                    (unwired) dbl[] [] ("History Data")
                    n2575 = local write "Engage"(FALSE ("Engage")) -> ()
                    n2576 = local write "RUN"(TRUE ("RUN")) -> ()
                    n2577 = local read "Humidity ( %RH )"() -> (→"Rh Before":dbl)
                  }
                }
                n2578 = local read "Test \nStatus"() -> (w3044:bool)
                n2579 = Select(t=w3042, s=w3044, f=0.0) -> (s? t:f=w3043:dbl)
                n2580 = local write "Frequency ( Hz )"(w3043) -> ()
              }
              frame #1 {
                w3134 = 1000000.0 ("x")
                # "HC;1/0\nST;VALUE"
                # "Elapsed time\ncof\nstroke\nAir temp\nTemp\nHumidity"
                # "acq timer\n\nact save time"
                # "convert to microseconds"
                n2581 = local read "COUNT"() -> (w3117:i32)
                n2582 = local read "Rate"() -> (w3130:dbl)
                n2583 = Divide(x=w3134, y=w3130) -> (x/y=w3135:dbl)
                n2584 = Greater Or Equal?(x=w3117, y=250) -> (x >= y?=w3116:bool)
                n2585 = Get Date/Time In Seconds() -> (seconds since 1Jan1904=w3137:timestamp)
                n2586 = case shown="True" w3116 {
                  frame False {
                    n2587 = local read "COUNT"() -> (w3138:i32)
                    n2588 = Increment(x=w3138) -> (x+1=w3139:i32)
                    n2589 = local write "COUNT"(w3139) -> ()
                  }
                  frame True {
                    n2590 = local write "COUNT"(0 ("COUNT")) -> ()
                  }
                }
                n2591 = local read "Samplingtime 2"() -> (w3115:dbl)
                n2592 = local read "act save time"() -> (w3132:dbl)
                n2593 = Divide(x=w3135, y=w3134) -> (x/y=w3133:dbl)
                n2594 = To Double Precision Float(number=w3137) -> (double precision float=w3126:dbl)
                n2595 = Add(x=w3132, y=w3115) -> (x+y=w3131:dbl)
                n2596 = local read "acq timer"() -> (w3136:dbl)
                n2597 = local read "COUNT"() -> (w3119:i32)
                n2598 = Greater Or Equal?(x=w3126, y=w3131) -> (x >= y?=w3114:bool)
                n2599 = Multiply(x=w3133, y=w3119) -> (x*y=w3125:dbl)
                n2600 = Subtract(x=w3126, y=w3136) -> (x-y=w3128:dbl)
                n2601 = local read "Save"() -> (w3129:bool)
                n2602 = Add(x=w3128, y=w3125) -> (x+y=w3112:dbl)
                "Elapsed time 3" <- w3112
                n2603 = And(x=w3114, y=w3129) -> (x .and. y?=w3127:bool)
                n2604 = Divide(x=w3112, y=60.0) -> (x/y=w3123:dbl)
                n2605 = local read "Test \nStatus"() -> (w3113:bool)
                n2606 = local read "clk"() -> (w3120:dbl)
                n2607 = Equal?(x=w3120, y=10.0) -> (x = y?=w3122:bool)
                n2608 = case shown="True" w3127 {
                  tunnel: w3126 -> [_ w3259]
                  tunnel: [FALSE ("Boolean 2") TRUE ("Boolean 2")] -> _
                  frame False {
                  }
                  frame True {
                    w3213 = ";" ("Substring")
                    # "Pid out/\nFreq response value"
                    n2609 = local write "act save time"(w3259) -> ()
                    n2610 = local read "FILE"() -> (w3207:string)
                    n2611 = call "file check.vi"("file name in"=w3207) -> ("error out"=w3210:errorcluster, "file name out"=w3205:string)  [unwired: 9 in]
                    n2612 = local read "LVDT STROKE"() -> (w3202:dbl)
                    n2613 = local read "Add up Stroke"() -> (w3200:dbl)
                    n2614 = call "FILE PATH CREATION.vi"("error in"=w3210, "FILE NAME :"=w3205) -> ("FILE OUT"=w3208:path)  [unwired: 8 in, 1 out]
                    n2615 = local read "STROKE Initialize"() -> (w3195:bool)
                    n2616 = Concatenate Strings(w3205, ".dgf" ("Substring")) -> (w3209:string)
                    n2617 = Subtract(x=w3202, y=w3200) -> (x-y=w3201:dbl)
                    n2618 = Absolute Value(x=w3201) -> (abs(x)=w3198:dbl)
                    n2619 = local read "FF 2"() -> (→"Frictional Force ( N )" →"Frictional Force ( N )":dbl)
                    n2620 = Build Path(base path=w3208, name or relative path=w3209) -> (appended path=w3204:path)
                    n2621 = flat-sequence {
                      tunnel: w3198 -> [w3264]
                      tunnel: [w3263] -> w3196
                      tunnel: w3195 -> [w3261]
                      tunnel: [w3266] -> w3197
                      tunnel: w3196 -> [w3266]
                      frame #0 {
                        n2622 = call <vilib>:"Mean PtByPt.vi"("x"=w3264, "sample length"="STROKE FILTER", "initialize"=w3261) -> ("mean"=w3263:dbl)  [unwired: 1 in, 1 out]
                      }
                      frame #1 {
                        "STROKE Initialize" <- FALSE ("STROKE Initialize")
                      }
                    }
                    n2623 = local read "COF 2"() -> (w3218:dbl)
                    "Coefficient of Friction" <- w3218
                    "COF 4" <- w3218
                    "Coefficient of Friction" <- w3218
                    n2624 = local read "TEMP"() -> (w3221:dbl)
                    "Temperature ( Deg C )" <- w3221
                    n2625 = local read "Humidity ( %RH )"() -> (w3220:dbl)
                    "Humidity ( %RH ) 2" <- w3220
                    n2626 = local read "Frequency ( Hz )"() -> (w3227:dbl)
                    n2627 = local read "LVDT STROKE DISPLAY"() -> (w3199:dbl)
                    n2628 = local read "Elapsed time"() -> (w3252:dbl)
                    n2629 = local read "AIR TEMP"() -> (w3225:dbl)
                    n2630 = local read "PID-out"() -> (w3230:dbl)
                    n2631 = local write "Temperature ( Deg C )"(w3221) -> ()
                    n2632 = Number To Fractional String(number=w3199, width (-)=i16 9 ("precision (6)"), precision (6)=i16 6) -> (F-format string=w3245:string)  [unwired: 1 in]
                    n2633 = Number To Fractional String(number=w3225, width (-)=i16 9 ("precision (6)"), precision (6)=i16 3) -> (F-format string=w3244:string)  [unwired: 1 in]
                    n2634 = Number To Fractional String(number=w3221, width (-)=i16 9 ("precision (6)"), precision (6)=i16 3) -> (F-format string=w3241:string)  [unwired: 1 in]
                    n2635 = Number To Fractional String(number=w3220, width (-)=i16 9 ("precision (6)"), precision (6)=i16 3) -> (F-format string=w3238:string)  [unwired: 1 in]
                    n2636 = Number To Fractional String(number=0.0, width (-)=i16 9 ("precision (6)"), precision (6)=i16 3) -> (F-format string=w3235:string)  [unwired: 1 in]